vi "GPU tracking demo.vi"() -> ()   [LabVIEW 2014]
uses:
  <vilib>/Native 3D Graph/xcontrol/3DPC_SurfacePlot.xctl
  <vilib>/Native 3D Graph/classes/Line/Line.lvclass
panel:
  out "Array of cal clusters 2":T1(array[cluster])
  out "subarray":sgl[](array[numeric])
  out "Array":dbl[](array[numeric])
  in  "use CPU?":bool
  in  "milliseconds to wait between frames in playback":u32=20
  out "XYZ Positions from GPU tracking program":refnum<class "Base Datatype.lvclass">[](xcontrol)
  out "Radial Intensity":dbl[](graph)=[131.39500427246094, 128.96400451660156, 128.37403869628906, 126.82691955566406, 124.55764770507812, 123.4681167602539, 119.52912902832031, 116.24790954589844, 111.82624053955078, 106.7735366821289, 102.0106430053711, 96.69518280029297, 91.58846282958984, 86.88774871826172, 82.81334686279297, 80.6859359741211, 80.26095581054688, 81.46810913085938, 85.67619323730469, 91.95333862304688, 100.05619812011719, 109.2582015991211, 118.6558837890625, 126.50748443603516, 132.62503051757812, 135.06956481933594, 133.0341796875, 127.21044158935547, 117.63623809814453, 107.00247955322266, 97.23945617675781, 90.6600341796875, 88.76422119140625, 92.13359832763672, 100.23995208740234, 110.32723236083984, 119.76548767089844, 125.3132553100586, 125.23900604248047, 119.34789276123047, 109.84239959716797, 100.73270416259766, 95.49577331542969, 95.76103210449219, 101.52030181884766, 109.9103012084961, 117.194580078125, 119.70499420166016, 116.30261993408203, 109.51485443115234, 102.31725311279297, 99.10395050048828, 101.57841491699219, 107.60005187988281, 113.52316284179688, 115.5927505493164, 112.95392608642578, 107.37324523925781, 102.9076156616211, 102.66129302978516]
  out "Frames from video files":T2(plugin-control)
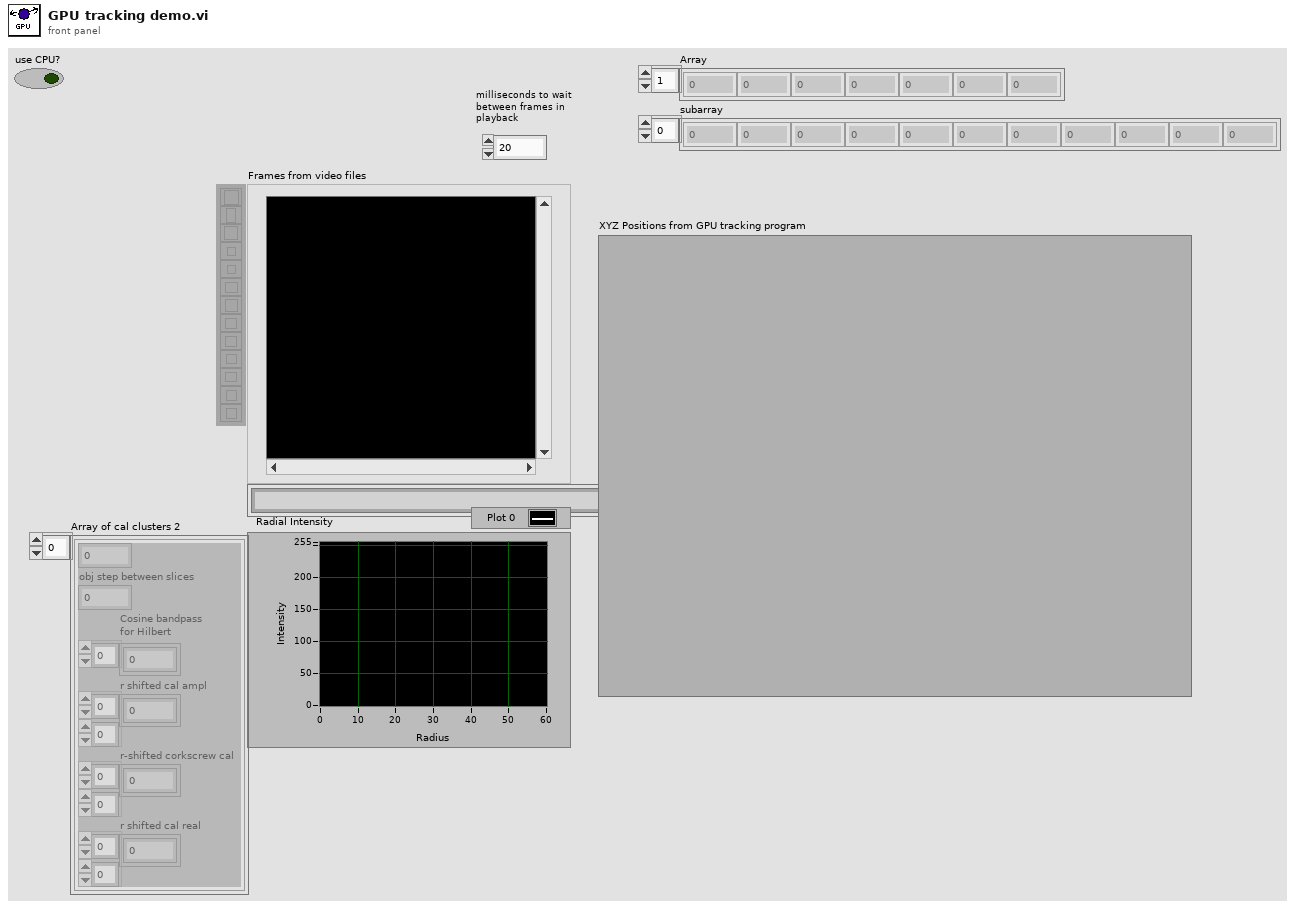
[diagram p1: front panel]
types:
  T1 = cluster{i32, "obj step between slices":dbl, "Cosine bandpass\nfor Hilbert":dbl[], "r shifted cal ampl":dbl[][], "r-shifted corkscrew cal":cdb[][], "r shifted cal real":dbl[][]}[]
  T2 = typedef "IMAQ Image.ctl" = refnum<image>
  T3 = cluster{"x,y pos array":sgl[][], "cal image array":sgl[][][], "# slices in stack":i32, "bandpass/forget array":i32[][], "obj step between slices":sgl, "# avg per slice":i32, "Date and time":string, "exp/ref array":i32[], "Pixel distance":sgl}
  T4 = typedef "Image Type" = u32
  T5 = cluster{i32, "obj step between slices":dbl, "Cosine bandpass\nfor Hilbert":dbl[], "r shifted cal ampl":dbl[][], "r-shifted corkscrew cal":cdb[][], "r shifted cal real":dbl[][]}
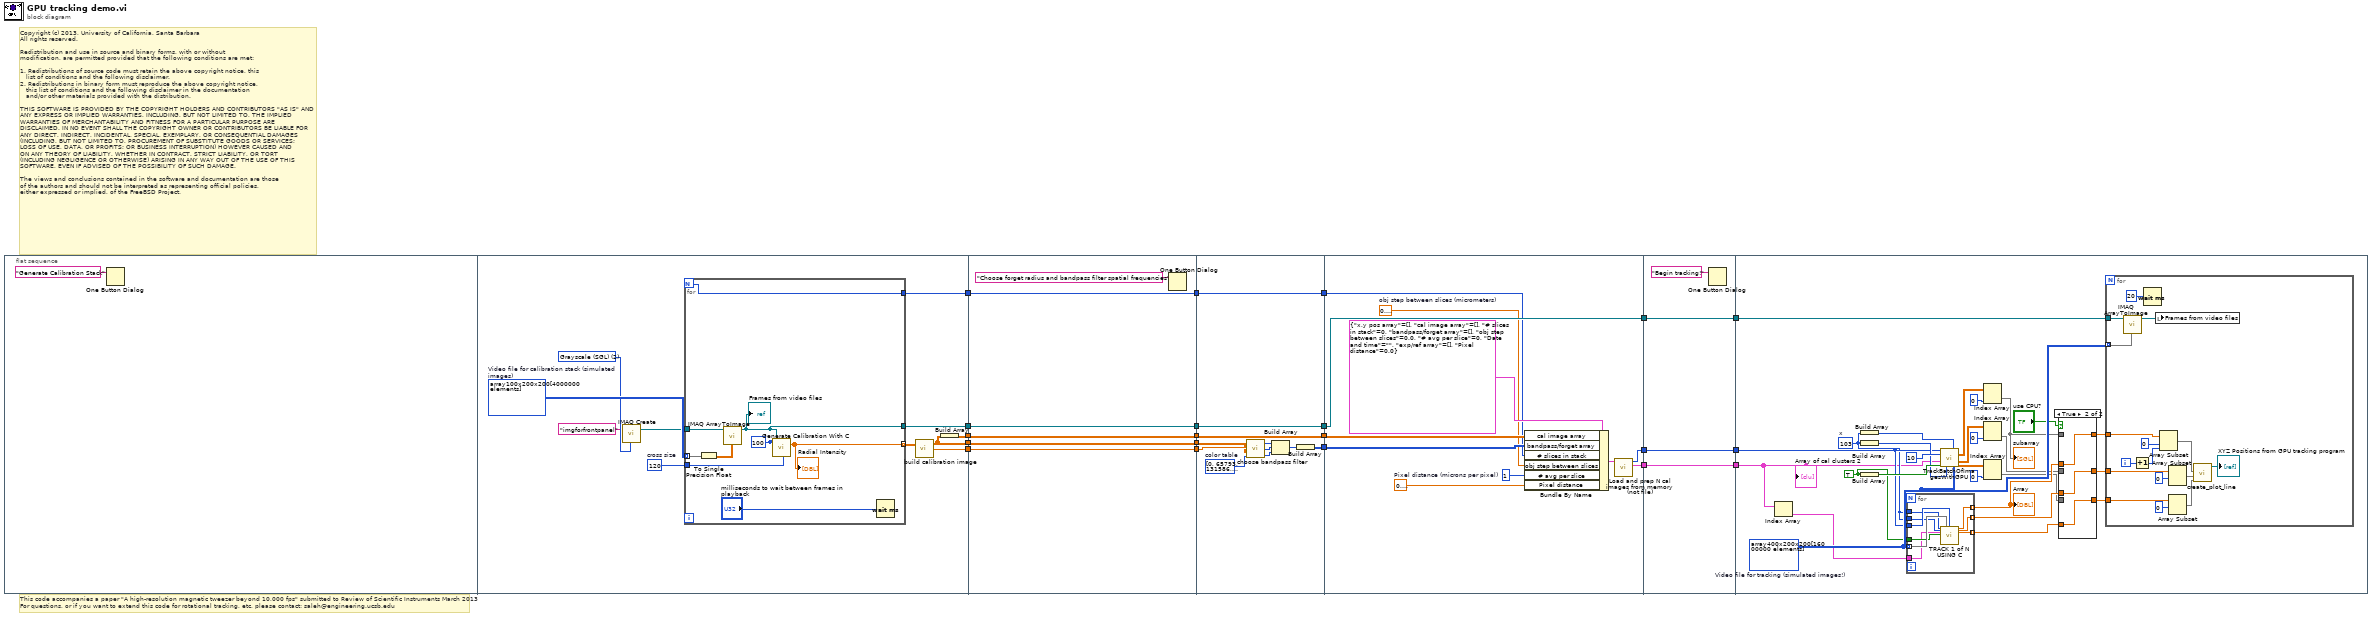
[diagram p0: block diagram]
diagram:
  # "Copyright (c) 2013, University of California, Santa Barbara\nAll rights reserved.\n\nRedistribution and use in source and binary forms, with or without\nmodification, are permitted provided that the following conditions are met: \n\n1. Redistributions of source code must retain the above copyright notice, this\n   list of conditions and the following disclaimer. \n2. Redistributions in binary form must reproduce the above copyright notice,\n   this list of conditions and the following disclaimer in the documentation\n   and/or other materials provided with the distribution. \n\nTHIS SOFTWARE IS PROVIDED BY THE COPYRIGHT HOLDERS AND CONTRIBUTORS \"AS IS\" AND\nANY EXPRESS OR IMPLIED WARRANTIES, INCLUDING, BUT NOT LIMITED TO, THE IMPLIED\nWARRANTIES OF MERCHANTABILITY AND FITNESS FOR A PARTICULAR PURPOSE ARE\nDISCLAIMED. IN NO EVENT SHALL THE COPYRIGHT OWNER OR CONTRIBUTORS BE LIABLE FOR\nANY DIRECT, INDIRECT, INCIDENTAL, SPECIAL, EXEMPLARY, OR CONSEQUENTIAL DAMAGES\n(INCLUDING, BUT NOT LIMITED TO, PROCUREMENT OF SUBSTITUTE GOODS OR SERVICES;\nLOSS OF USE, DATA, OR PROFITS; OR BUSINESS INTERRUPTION) HOWEVER CAUSED AND\nON ANY THEORY OF LIABILITY, WHETHER IN CONTRACT, STRICT LIABILITY, OR TORT\n(INCLUDING NEGLIGENCE OR OTHERWISE) ARISING IN ANY WAY OUT OF THE USE OF THIS\nSOFTWARE, EVEN IF ADVISED OF THE POSSIBILITY OF SUCH DAMAGE.\n\nThe views and conclusions contained in the software and documentation are those\nof the authors and should not be interpreted as representing official policies, \neither expressed or implied, of the FreeBSD Project."
  # "This code accompanies a paper \"A high-resolution magnetic tweezer beyond 10,000 fps\" submitted to Review of Scientific Instruments March 2013\nFor questions, or if you want to extend this code for rotational tracking, etc, please contact: saleh@engineering.ucsb.edu"
  n1 = flat-sequence {
    tunnel: [w24] -> w5
    tunnel: [w32] -> w4
    tunnel: [w22] -> w3
    tunnel: [w31] -> w2
    tunnel: [w30] -> w1
    tunnel: [w47] -> w10
    tunnel: [w46] -> w9
    tunnel: [w45] -> w8
    tunnel: [w44] -> w7
    tunnel: [w43] -> w6
    tunnel: w5 -> [w47]
    tunnel: w4 -> [w46]
    tunnel: w3 -> [w45]
    tunnel: w2 -> [w44]
    tunnel: w1 -> [w43]
    tunnel: [w58] -> w14
    tunnel: [w57] -> w13
    tunnel: [w48] -> w12
    tunnel: [w56] -> w11
    tunnel: w10 -> [w58]
    tunnel: w9 -> [w57]
    tunnel: w8 -> [w56]
    tunnel: w7 -> [w50]
    tunnel: w6 -> [w49]
    tunnel: [w69] -> w18
    tunnel: [w68] -> w17
    tunnel: [w67] -> w15
    tunnel: w14 -> [w69]
    tunnel: w13 -> [w64]
    tunnel: w12 -> [w63]
    tunnel: w11 -> [w61]
    tunnel: [w73] -> w20
    tunnel: [w71] -> w19
    tunnel: w18 -> [w73]
    tunnel: w17 -> [w71]
    tunnel: [w70] -> w16
    tunnel: w15 -> [w70]
    tunnel: w20 -> [w100]
    tunnel: w19 -> [w75]
    tunnel: w16 -> [w88]
    frame #0 {
      n2 = One Button Dialog(message="Generate Calibration Stack") -> ()  [unwired: 1 in, 1 out]
    }
    frame #1 {
      w28 = 120  # cross size
      w29 = u8[][][] array100x200x200[4000000 elements]  # Video file for calibration stack (simulated images)
      w27 = T4 2 items=["Grayscale (U8)", "Grayscale (I16)", "Grayscale (SGL)", "Complex (CSG)", "RGB (U32)", "HSL (U32)", "RGB (U64)", "Grayscale (U16)"] ("Image Type")
      n3 = call "IMAQ Create"("Image Name"="imgforfrontpanel", "Image Type"=w27) -> ("New Image"=w25:T2)  [unwired: 3 in, 1 out]
      n4 = for {
        N -> [w34]
        tunnel: w29 -> [w39] mode=indexing
        tunnel: w25 -> [w41]
        tunnel: w28 -> [w37]
        tunnel: [w35] -> w23 mode=indexing
        tunnel: [w34] -> w22
        tunnel: [w33] -> w24
        w38 = i16 100 ("starting x 1")
        n5 = To Single Precision Float(number=w39) -> (single precision float=w36:sgl[][])
        n6 = call "IMAQ ArrayToImage"("Image Pixels (Float)"=w36, "Image"=w41) -> ("Image Out"=w33:T2)  [unwired: 8 in, 1 out]
        "Frames from video files" <- w33
        n7 = call "Generate Calibration With C.vi"("starting x 1"=w38, "starting y 1"=w38, "Image"=w33, "cross size"=w37) -> ("radial intensity profile 1"=w35:dbl[])  [unwired: 21 in, 2 out]
        "Radial Intensity" <- w35
        n8 = Wait (ms)(milliseconds to wait="milliseconds to wait between frames in playback") -> ()  [unwired: 1 out]
      }
      n9 = call "build calibration image.vi"("1-sided cal image"=w23) -> ("2-sided cal image"=w30:dbl[][], "avg power spectrum of stack"=w31:dbl[])  [unwired: 2 in]
      n10 = Build Array(w30) -> (w32:dbl[][][])
    }
    frame #2 {
      n11 = One Button Dialog(message="Choose forget radius and bandpass filter spatial frequencies") -> ()  [unwired: 1 in, 1 out]
    }
    frame #3 {
      w55 = u32[] [0, 65793, 131586, 197379, 263172, 328965, 394758, 460551, 526344, 592137, 657930, 723723, 789516, 855309, 921102, 986895, 1052688, 1118481, 1184274, 1250067, 1315860, 1381653, 1447446, 1513239, 1579032, 1644825, 1710618, 1776411, 1842204, 1907997, 1973790, 2039583, 2105376, 2171169, 2236962, 2302755, 2368548, 2434341, 2500134, 2565927, 2631720, 2697513, 2763306, 2829099, 2894892, 2960685, 3026478, 3092271, 3158064, 3223857, 3289650, 3355443, 3421236, 3487029, 3552822, 3618615, 3684408, 3750201, 3815994, 3881787, 3947580, 4013373, 4079166, 4144959, 4210752, 4276545, 4342338, 4408131, 4473924, 4539717, 4605510, 4671303, 4737096, 4802889, 4868682, 4934475, 5000268, 5066061, 5131854, 5197647, 5263440, 5329233, 5395026, 5460819, 5526612, 5592405, 5658198, 5723991, 5789784, 5855577, 5921370, 5987163, 6052956, 6118749, 6184542, 6250335, 6316128, 6381921, 6447714, 6513507, 6579300, 6645093, 6710886, 6776679, 6842472, 6908265, 6974058, 7039851, 7105644, 7171437, 7237230, 7303023, 7368816, 7434609, 7500402, 7566195, 7631988, 7697781, 7763574, 7829367, 7895160, 7960953, 8026746, 8092539, 8158332, 8224125, 8289918, 8355711, 8421504, 8487297, 8553090, 8618883, 8684676, 8750469, 8816262, 8882055, 8947848, 9013641, 9079434, 9145227, 9211020, 9276813, 9342606, 9408399, 9474192, 9539985, 9605778, 9671571, 9737364, 9803157, 9868950, 9934743, 10000536, 10066329, 10132122, 10197915, 10263708, 10329501, 10395294, 10461087, 10526880, 10592673, 10658466, 10724259, 10790052, 10855845, 10921638, 10987431, 11053224, 11119017, 11184810, 11250603, 11316396, 11382189, 11447982, 11513775, 11579568, 11645361, 11711154, 11776947, 11842740, 11908533, 11974326, 12040119, 12105912, 12171705, 12237498, 12303291, 12369084, 12434877, 12500670, 12566463, 12632256, 12698049, 12763842, 12829635, 12895428, 12961221, 13027014, 13092807, 13158600, 13224393, 13290186, 13355979, 13421772, 13487565, 13553358, 13619151, 13684944, 13750737, 13816530, 13882323, 13948116, 14013909, 14079702, 14145495, 14211288, 14277081, 14342874, 14408667, 14474460, 14540253, 14606046, 14671839, 14737632, 14803425, 14869218, 14935011, 15000804, 15066597, 15132390, 15198183, 15263976, 15329769, 15395562, 15461355, 15527148, 15592941, 15658734, 15724527, 15790320, 15856113, 15921906, 15987699, 16053492, 16119285, 16185078, 16250871, 16316664, 16382457, 16448250, 16514043, 16579836, 16645629, 16711422, 16777215]  # color table
      n12 = call "choose bandpass filter.vi"("color table"=w55, "Cal image data"=w49, "Power spectrum"=w50) -> ("forget radius"=w51:i32, "High bandpass"=w52:i32, "Low bandpass"=w53:i32)  [unwired: 1 in]
      n13 = Build Array(w53, w52, w51) -> (w54:i32[])
      n14 = Build Array(w54) -> (w48:i32[][])
    }
    frame #4 {
      w59 = sgl 0.1  # Pixel distance (microns per pixel)
      w60 = sgl 0.1  # obj step between slices (micrometers)
      n15 = Bundle By Name(cluster=T3 {"x,y pos array"=[], "cal image array"=[], "# slices in stack"=0, "bandpass/forget array"=[], "obj step between slices"=0.0, "# avg per slice"=0, "Date and time"="", "exp/ref array"=[], "Pixel distance"=0.0} ("input cluster"), "cal image array"=w64, "bandpass/forget array"=w63, "# slices in stack"=w61, "obj step between slices"=w60, "# avg per slice"=1, "Pixel distance"=w59) -> (w62:T3)
      n16 = call "Load and prep N cal images from memory (not file).vi"("data"=w62) -> ("Array of cal clusters 2"=w68:T1, "cross size"=w67:i32)  [unwired: 5 in, 4 out]
    }
    frame #5 {
      n17 = One Button Dialog(message="Begin tracking!") -> ()  [unwired: 1 in, 1 out]
    }
    frame #6 {
      w77 = TRUE ("Normalize?")
      w76 = 103  # x
      w89 = u8[][][] array400x200x200[16000000 elements]  # Video file for tracking (simulated images!)
      n18 = Index Array(array=w75) -> (element=w74:T5)  [unwired: 1 in]
      n19 = Build Array(w76) -> (w90:i32[])
      n20 = Build Array(w76) -> (w91:i32[])
      n21 = Build Array(w77) -> (w92:bool[])
      n22 = for {
        tunnel: w89 -> [w115] mode=indexing
        tunnel: w88 -> [w114]
        tunnel: [w113] -> w87 mode=indexing
        tunnel: [w112] -> w86 mode=indexing
        tunnel: [w111] -> w85 mode=indexing
        tunnel: w77 -> [w110]
        tunnel: w76 -> [w109]
        tunnel: w76 -> [w108]
        tunnel: w74 -> [w107]
        n23 = call "TRACK 1 of N USING C.vi"("starting x 1"=w108, "starting y 1"=w109, "Calibration cluster 1"=w107, "Bead 1 is good? in"=w110, "Image Pixels (Float)"=w115, "cross size"=w114) -> ("X pos 1"=w113:dbl, "Y pos 1"=w112:dbl, "Z pos 1"=w111:dbl)  [unwired: 16 in, 3 out]
      }
      "Array" <- w87
      n24 = call "TrackBatchOfImagesWithGPU.vi"("cross size"=w88, "X Array Input"=w90, "Cross Thickness"=10, "Array Calibration Cluster"=w75, "Bead Is Good IN"=w92, "Y Array Input"=w91, "Array of Images"=w89) -> ("GPU tracking X"=w95:sgl[][], "Y Output from GPU"=w94:sgl[][], "Z from gpu"=w93:sgl[][])  [unwired: 4 in, 2 out]
      n25 = Index Array(array=w95, index (col)=0 ("disabled index (col)")) -> (element=w84:sgl[])  [unwired: 1 in]
      "subarray" <- w84
      n26 = Index Array(array=w94, index (col)=0 ("disabled index (col)")) -> (element=w83:sgl[])  [unwired: 1 in]
      n27 = Index Array(array=w93, index (col)=0 ("disabled index (col)")) -> (element=w82:sgl[])  [unwired: 1 in]
      n28 = case shown="True" "use CPU?" {
        tunnel: w87 -> [_ w106]
        tunnel: w86 -> [_ w105]
        tunnel: w85 -> [_ w104]
        tunnel: [w103 w106] -> w81
        tunnel: [w102 w105] -> w80
        tunnel: [w101 w104] -> w79
        tunnel: w84 -> [w103 _]
        tunnel: w83 -> [w102 _]
        tunnel: w82 -> [w101 _]
        frame False {
        }
        frame True {
        }
      }
      n29 = for {
        tunnel: w100 -> [w130]
        tunnel: w89 -> [w129] mode=indexing
        tunnel: w81 -> [w121]
        tunnel: w80 -> [w120]
        tunnel: w79 -> [w119]
        i -> [w126]
        n30 = call "IMAQ ArrayToImage"("Image Pixels (Float)"=w129, "Image"=w130) -> ("Image Out"=w131:T2)  [unwired: 8 in, 1 out]
        n31 = Increment(x=w126) -> (x+1=w125:i32)
        n32 = Wait (ms)(milliseconds to wait=u32 20) -> ()  [unwired: 1 out]
        n33 = local write "Frames from video files"(w131) -> ()
        n34 = Array Subset(array=w121, index=0, length=w125) -> (w118:dbl[])
        n35 = Array Subset(array=w120, index=0) -> (w117:dbl[])  [unwired: 1 in]
        n36 = Array Subset(array=w119, index=0) -> (w116:dbl[])  [unwired: 1 in]
        n37 = call <vilib>:"create_plot_line.vi"("z vector"=w116, "y vector"=w117, "x vector"=w118) -> ("plots out"=→"XYZ Positions from GPU tracking program":refnum<class "Base Datatype.lvclass">[])  [unwired: 2 in, 6 out]
      }
      "Array of cal clusters 2" <- w75
    }
  }
